vi "15-12-13 UHR-Fleezers Control (host) - 15.2.1UCB Darwin.vi"() -> ()   [LabVIEW 2014] (continued)
          tunnel: w1189 -> [_]
          tunnel: "Center Y Frequency (MHz)" -> [w1283]
          shift-right: [w1244] -> _
          shift-left: w1184 -> [w1251]
          shift-right: [w1242] -> _
          shift-left: w1184 -> [w1250]
          shift-right: [w1235] -> _
          shift-left: w1184 -> [w1248]
          shift-right: [w1233] -> _
          shift-left: w1184 -> [w1247]
          tunnel: "Move in a Circle" -> [_]
          tunnel: ["Back to start on finish?"] -> w1188
          tunnel: w1186 -> [_]
          tunnel: w1185 -> [w1265]
          tunnel: w1184 -> [w1246]
          shift-right: [w1217] -> _
          shift-left: 0.0 -> [w1215]
          i -> [w1224]
          stop <- w1288 stop-if-true
          w1232 = 0 ("index")
          w1253 = 1 ("dimension size")
          # "Keep phase within\n2pi so errors don't \nbuild"
          # "Accumulated\nphase"
          # "Current phase"
          # "Trap 2"
          # "Trap 1"
          # "ignore if N = 0"
          # "r"
          # "r"
          # "r"
          # "r"
          # "\"omega*t\""
          # "Trap 2"
          # "Trap separation (radians)"
          # "Trap 1"
          # "Offset (starts\n at bottom of\n the circle)"
          # "omega"
          n764 = node-c288() -> (w1301:i64)  [unwired: 1 in]
          n765 = Divide(x=w1301, y=1000) -> (x/y=w1220:dbl)
          n766 = Divide(x="2D Motion Trap Separation (MHz)", y="Radius (MHz)") -> (x/y=w1275:dbl)
          n767 = Negate(x=w1220) -> (-x=w1219:dbl)
          n768 = Divide(x="Trap 2 phase shift (deg)", y=360.0) -> (x/y=w1266:dbl)
          n769 = Inverse Sine(1:w1275) -> (0:w1211:dbl)
          n770 = Multiply(x=6.283185307179586, y=w1266) -> (x*y=w1212:dbl)
          n771 = Multiply(x=6.283185307179586, y="2D Motion Frequency (Hz)") -> (x*y=w1223:dbl)
          n772 = Select(t=w1220, s="Counterclockwise/Clockwise", f=w1219) -> (s? t:f=w1222:dbl)
          n773 = Multiply(x=w1223, y=w1222) -> (x*y=w1213:dbl)
          n774 = Select(t=w1211, s="Trap shift\nmethod", f=w1212) -> (s? t:f=w1210:dbl)
          n775 = Add(x=w1213, y=w1215) -> (x+y=w1216:dbl)
          n776 = Add(x=w1216, y=w1210) -> (x+y=w1272:dbl)
          n777 = Add(x=w1216, y=1.5707963267948966) -> (x+y=w1221:dbl)
          n778 = Add(x=w1272, y=1.5707963267948966) -> (x+y=w1285:dbl)
          n779 = Cosine(x=w1221) -> (cos(x)=w1299:dbl)
          n780 = Sine(x=w1221) -> (sin(x)=w1298:dbl)
          n781 = Multiply(x=w1299, y="Radius (MHz)") -> (x*y=w1292:dbl)
          n782 = Cosine(x=w1285) -> (cos(x)=w1297:dbl)
          n783 = Sine(x=w1285) -> (sin(x)=w1296:dbl)
          n784 = Multiply(x=w1298, y="Radius (MHz)") -> (x*y=w1291:dbl)
          n785 = Multiply(x=w1297, y="Radius (MHz)") -> (x*y=w1295:dbl)
          n786 = Multiply(x=w1296, y="Radius (MHz)") -> (x*y=w1293:dbl)
          n787 = Add(x=w1292, y=w1290) -> (x+y=w1241:dbl)
          n788 = Add(x=w1291, y=w1283) -> (x+y=w1239:dbl)
          n789 = Greater Or Equal?(x=w1224, y="N steps then stop") -> (x >= y?=w1282:bool)
          n790 = Add(x=w1295, y=w1294) -> (x+y=w1230:dbl)
          n791 = Add(x=w1293, y=w1283) -> (x+y=w1228:dbl)
          n792 = Not Equal To 0?(x="N steps then stop") -> (x != 0?=w1278:bool)
          n793 = And(x=w1282, y=w1278) -> (x .and. y?=w1279:bool)
          n794 = local read "Trap 1 sum mean"() -> (w1262:dbl)
          n795 = local read "Stop All"() -> (w1287:bool)
          n796 = local write "BD 1 Frequency 1 (MHz)"(w1241) -> ()
          n797 = local write "BD 2 Frequency 1 (MHz)"(w1239) -> ()
          n798 = local write "BD 1 Frequency 2 (MHz)"(w1230) -> ()
          n799 = local write "BD 2 Frequency 2 (MHz)"(w1228) -> ()
          n800 = Select(t=w1224, s="test", f=w1262) -> (s? t:f=→"Waveform Chart":dbl)
          n801 = Compound Arithmetic op=OR(w1287, "Stop Moving", w1279) -> (w1288:bool)
          n802 = local read "BD 1 Frequency 3 (MHz)"() -> (w1271:dbl)
          n803 = local read "BD 2 Frequency 3 (MHz)"() -> (w1270:dbl)
          n804 = Select(t=w1246, s="Reset graph", f=w1247) -> (s? t:f=w1227:dbl[])
          n805 = Select(t=w1246, s="Reset graph", f=w1248) -> (s? t:f=w1229:dbl[])
          n806 = Select(t=w1246, s="Reset graph", f=w1250) -> (s? t:f=w1238:dbl[])
          n807 = Select(t=w1246, s="Reset graph", f=w1251) -> (s? t:f=w1240:dbl[])
          n808 = Initialize Array(w1228, w1253) -> (w1254:dbl[])
          n809 = Initialize Array(w1239, w1253) -> (w1257:dbl[])
          n810 = Initialize Array(w1230, w1253) -> (w1255:dbl[])
          n811 = Initialize Array(w1241, w1253) -> (w1258:dbl[])
          n812 = local read "Y RF Frequency Limits (MHz)"() -> (w1268:T18)
          n813 = local read "X RF Frequency Limits (MHz)"() -> (w1269:T18)
          n814 = call "set RF board frequency - interlace.vi"("Board 2 Frequency Limits"=w1268, "Board 1 Frequency Limits"=w1269, "FPGA VI Reference In"=w1265, "Board 2 Frequency 3 (MHz)"=w1270, "Board 1 Frequency 3 (MHz)"=w1271, "Board 2 Frequency 2 (MHz)"=w1228, "Board 2 Frequency 1 (MHz)"=w1239, "Board 1 Frequency 2 (MHz)"=w1230, "Board 1 Frequency 1  (MHz)"=w1241) -> ()  [unwired: 1 in, 2 out]
          n815 = Bundle(w1255, w1254) -> (w1226:cluster{dbl[], dbl[]})  [unwired: 1 in]
          n816 = Bundle(w1258, w1257) -> (w1256:cluster{dbl[], dbl[]})  [unwired: 1 in]
          n817 = Build Array (concatenate)(w1241, w1240) -> (w1245:dbl[])
          n818 = Build Array (concatenate)(w1239, w1238) -> (w1243:dbl[])
          n819 = Build Array (concatenate)(w1230, w1229) -> (w1236:dbl[])
          n820 = Build Array (concatenate)(w1228, w1227) -> (w1234:dbl[])
          n821 = Bundle(w1245, w1243) -> (w1225:cluster{dbl[], dbl[]})  [unwired: 1 in]
          n822 = Bundle(w1236, w1234) -> (w1252:cluster{dbl[], dbl[]})  [unwired: 1 in]
          n823 = Build Array(w1256, w1226, w1225, w1252) -> (→"Trap trajectories":cluster{dbl[], dbl[]}[])
          n824 = case "To pause the process" shown="True" "Pause rotation" {
            frame False {
            }
            frame True {
              n825 = while {
                stop <- w1304 stop-if-true
                n826 = local read "Pause rotation"() -> (w1305:bool)
                n827 = Wait (ms)(milliseconds to wait=u32 10) -> ()  [unwired: 1 out]
                n828 = Not(x=w1305) -> (.not. x?=w1304:bool)
              }
            }
          }
          n829 = Decrement(x="N steps to plot") -> (x-1=w1231:i32)
          n830 = Array Subset(array=w1243, index=w1232, length=w1231) -> (w1242:dbl[])
          n831 = Array Subset(array=w1245, index=w1232, length=w1231) -> (w1244:dbl[])
          n832 = Array Subset(array=w1236, index=w1232, length=w1231) -> (w1235:dbl[])
          n833 = Array Subset(array=w1234, index=w1232, length=w1231) -> (w1233:dbl[])
          n834 = Quotient & Remainder(x=w1216, y=6.283185307179586) -> (x-y*floor(x/y)=w1217:dbl)  [unwired: 1 out]
          n835 = node-c288() -> ()  [unwired: 1 in, 1 out]
        }
        n836 = node-c288(w1197) -> ()  [unwired: 1 out]
        n837 = case shown="True" w1188 {
          tunnel: w1192 -> [_ w1203]
          tunnel: w1191 -> [_ w1202]
          tunnel: w1190 -> [_ w1201]
          tunnel: w1189 -> [_ w1200]
          frame False {
          }
          frame True {
            n838 = flat-sequence {
              tunnel: w1203 -> [w1207]
              tunnel: w1202 -> [w1206]
              tunnel: w1201 -> [w1205]
              tunnel: w1200 -> [w1204]
              frame #0 {
                n839 = local write "BD 1 Frequency 1 (MHz)"(w1207) -> ()
                n840 = local write "BD 2 Frequency 1 (MHz)"(w1206) -> ()
                n841 = local write "BD 1 Frequency 2 (MHz)"(w1205) -> ()
                n842 = local write "BD 2 Frequency 2 (MHz)"(w1204) -> ()
              }
              frame #1 {
                n843 = property on="Update all trap values" class="Bool (strict)"("Val(Sgnl)"=TRUE ("Value (Signaling)")) -> ()  [unwired: 2 in, 2 out]
              }
            }
          }
        }
      }
      event "Stop All": Value Change {
        # "Stopping blue laser before shutting off program"
        n844 = event-data() -> ()  [unwired: 1 in, 5 out]
        n845 = local read "Delay (ms)"() -> (w1315:i32)
        n846 = call "serial write macro.vi"("String"="l0", "Delay (ms)"=w1315, "VISA resource name"=w1318) -> ("read buffer"=w1313:string, "error out"=w1314:errorcluster, "VISA resource name out"=w1317:refnum<visa-resource-name>)
        n847 = local write "read blue buffer"(w1313) -> ()
        n848 = local write "Blue Error Out"(w1314) -> ()
        n849 = VISA Close(VISA resource name=w1317) -> ()  [unwired: 1 in, 1 out]
        n850 = local read "Stop All"() -> (w1319:bool)
      }
      event "Sensitivity", "Offset Current Sign", "Offset Current Value", "Offset Current", "Bias Voltage", "Bias Voltage (mV)", "Filter Type", "Lowpass 3dB Point", "Highpass 3dB Point", "Filter Reset", "Invert Signal", "Gain Mode", "Send Command": Value Change {
        w1326 = 250 ("Delay (ms)")
        n851 = event-data() -> ()  [unwired: 1 in, 5 out]
        n852 = event shown="[0] \"Sensitivity\": Value Change" {
          selector: _ -> [_ _ _ _ _ _ _ _ _ _ _ _ _]
          dyn-events: _ -> [_ _ _ _ _ _ _ _ _ _ _ _ _]
          timeout: _ -> [_ _ _ _ _ _ _ _ _ _ _ _ _]
          tunnel: [w1338 w1346 w1354 w1363 w1373 w1381 w1384 w1388 w1391 w1394 w1397 w1404 "Command"] -> w1325
          tunnel: [w1333 w1340 w1350 w1357 w1367 w1377 _ _ _ _ _ w1400 _] -> w1320
          event "Sensitivity": Value Change {
            n853 = event-data() -> ()  [unwired: 1 in, 5 out]
            n854 = property on="Sensitivity" class="CmbBox"() -> ("Value"=→"Gain":string)  [unwired: 2 in, 2 out]
            n855 = Concatenate Strings("SENS ", "Sensitivity") -> (w1338:string)
            n856 = local read "Gain"() -> (w1335:string)
            n857 = Concatenate Strings("gain set at ", w1335) -> (w1333:string)
          }
          event "Offset Current Sign": Value Change {
            n858 = event-data() -> ()  [unwired: 1 in, 4 out]
            n859 = Boolean To (0,1)(Boolean="Offset Current Sign") -> (0, 1=w1349:i16)
            n860 = Select(t="positive", s="Offset Current Sign", f="negative") -> (s? t:f=w1341:string)
            n861 = Number To Decimal String(number=w1349) -> (decimal integer string=w1348:string)  [unwired: 1 in]
            n862 = Concatenate Strings("IOSN " ("string"), w1348) -> (w1346:string)
            n863 = Concatenate Strings("offset current sign ", w1341) -> (w1340:string)
          }
          event "Offset Current Value": Value Change {
            n864 = event-data() -> ()  [unwired: 1 in, 5 out]
            n865 = property on="Offset Current Value" class="CmbBox"() -> ("Value"=→"Read offset current":string)  [unwired: 2 in, 2 out]
            n866 = local read "Read offset current"() -> (w1351:string)
            n867 = Concatenate Strings("IOLV ", "Offset Current Value") -> (w1354:string)
            n868 = Concatenate Strings("offset current value ", w1351) -> (w1350:string)
          }
          event "Offset Current": Value Change {
            n869 = event-data() -> ()  [unwired: 1 in, 5 out]
            n870 = Boolean To (0,1)(Boolean="Offset Current") -> (0, 1=w1366:i16)
            n871 = Select(t="on", s="Offset Current", f="off") -> (s? t:f=w1358:string)
            n872 = Number To Decimal String(number=w1366) -> (decimal integer string=w1365:string)  [unwired: 1 in]
            n873 = Concatenate Strings("IOON " ("string"), w1365) -> (w1363:string)
            n874 = Concatenate Strings("offset current ", w1358) -> (w1357:string)
          }
          event "Bias Voltage": Value Change {
            n875 = event-data() -> ()  [unwired: 1 in, 5 out]
            n876 = Boolean To (0,1)(Boolean="Bias Voltage") -> (0, 1=w1374:i16)
            n877 = Number To Decimal String(number=w1374) -> (decimal integer string=w1375:string)  [unwired: 1 in]
            n878 = Select(t="on", s="Bias Voltage", f="off") -> (s? t:f=w1368:string)
            n879 = Concatenate Strings("BSON " ("string"), w1375) -> (w1373:string)
            n880 = Concatenate Strings("bias voltage", w1368) -> (w1367:string)
          }
          event "Bias Voltage (mV)": Value Change {
            n881 = event-data() -> ()  [unwired: 1 in, 5 out]
            n882 = Number To Decimal String(number="Bias Voltage (mV)") -> (decimal integer string=w1383:string)  [unwired: 1 in]
            n883 = Number To Fractional String(number="Bias Voltage (mV)") -> (F-format string=w1378:string)  [unwired: 3 in]
            n884 = Concatenate Strings("BSLV " ("string"), w1383) -> (w1381:string)
            n885 = Concatenate Strings("bias voltage value ", w1378) -> (w1377:string)
          }
          event "Filter Type": Value Change {
            n886 = event-data() -> ()  [unwired: 1 in, 5 out]
            n887 = Concatenate Strings("FLTT " ("string"), "Filter Type") -> (w1384:string)
          }
          event "Lowpass 3dB Point": Value Change {
            n888 = event-data() -> ()  [unwired: 1 in, 5 out]
            n889 = Concatenate Strings("LFRQ " ("string"), "Lowpass 3dB Point") -> (w1388:string)
          }
          event "Highpass 3dB Point": Value Change {
            n890 = event-data() -> ()  [unwired: 1 in, 5 out]
            n891 = Concatenate Strings("HFRQ " ("string"), "Highpass 3dB Point") -> (w1391:string)
          }
          event "Filter Reset": Value Change {
            n892 = event-data() -> ()  [unwired: 1 in, 5 out]
            n893 = Select(t="ROLD", s="Filter Reset", f="") -> (s? t:f=w1394:string)
          }
          event "Gain Mode": Value Change {
            n894 = event-data() -> ()  [unwired: 1 in, 5 out]
            n895 = Concatenate Strings("GNMD " ("string"), "Gain Mode") -> (w1397:string)
          }
          event "Invert Signal": Value Change {
            n896 = event-data() -> ()  [unwired: 1 in, 5 out]
            n897 = Boolean To (0,1)(Boolean="Invert Signal") -> (0, 1=w1407:i16)
            n898 = Number To Decimal String(number=w1407) -> (decimal integer string=w1406:string)  [unwired: 1 in]
            n899 = Concatenate Strings("INVT " ("string"), w1406) -> (w1404:string)
            n900 = Select(t="signal inverted", s="Invert Signal", f="signal not inverted") -> (s? t:f=w1400:string)
          }
          event "Send Command": Value Change {
            n901 = event-data() -> ()  [unwired: 1 in, 5 out]
          }
        }
        "Command Sent" <- w1325
        n902 = local read "Save Event Log?"() -> (w1321:bool)
        n903 = local read "Saving..."() -> (w1322:bool)
        n904 = And(x=w1321, y=w1322) -> (x .and. y?=w1323:bool)
        n905 = case shown="True" w1323 {
          tunnel: w1320 -> [_ w1330]
          frame False {
          }
          frame True {
            n906 = local read "Time (s)"() -> (w1331:dbl)
            n907 = local read "log file ref"() -> (w1332:refnum<file>)
            n908 = call "write to event log.vi"("log file ref"=w1332, "time"=w1331, "input string"=w1330) -> ()  [unwired: 8 in]
          }
        }
        n909 = call "preamp serial write macro.vi"("String"=w1325, "Delay (ms)"=w1326, "VISA resource name"=w1329) -> ("read buffer"=→"Reply":string, "error out"=w1328:errorcluster)  [unwired: 1 out]
        n910 = call "preamp serial write macro.vi"("String"=w1325, "Delay (ms)"=w1326, "VISA resource name"=w1324) -> ()  [unwired: 3 out]
        n911 = local write "Preamp Error Out"(w1328) -> ()
      }
    }
    n912 = node-c288() -> ()  [unwired: 1 in, 1 out]
  }
  n913 = node-c288() -> (w27:T27)  [unwired: 4 out]
  n914 = node-c288(2 ("Processor")) -> (w59:T27)  [unwired: 3 out]
  n915 = disable-structure shown="Disabled" {
    frame Disabled {
      n916 = while "Duncan's play event loop" {
        stop <- w1411 stop-if-true
        n917 = Create User Event(user event datatype=TRUE ("Boolean")) -> (user event=w1412:refnum<user-event>)  [unwired: 1 in, 1 out]
        n918 = Create User Event(user event datatype=TRUE ("Boolean")) -> (user event=w1418:refnum<user-event>)  [unwired: 1 in, 1 out]
        n919 = global write "Global for fluorescence simulation mean (30 samples), (power series).vi" "Red Signal"(w1412) -> ()
        n920 = global write "Global for fluorescence simulation mean (30 samples), (power series).vi" "Green Signal"(w1418) -> ()
        n921 = register-events(w1418, w1412) -> (reference out=w1417:refnum<event-registration>)  [unwired: 2 in, 1 out]
        n922 = event shown="[1] \"Start assembly line\": Value Change" {
          selector: w1417 -> [_ _ _ _]
          dyn-events: _ -> [_ _ _ _]
          timeout: 100 -> [_ _ _ _]
          event Timeout {
            n923 = event-data() -> ()  [unwired: 1 in, 2 out]
          }
          event "Start assembly line": Value Change {
            n924 = event-data() -> ("OldVal"=w1420:bool)  [unwired: 1 in, 4 out]
            n925 = case shown="True" w1420 {
              selector: w1420 -> [_ w1421]
              frame False {
              }
              frame True {
                n926 = property on="Move to Position 3" class="Bool"("Val(Sgnl)"=w1421) -> ()  [unwired: 2 in, 2 out]
                n927 = case shown="1" "Numeric" {
                  frame 0, Default {
                  }
                  frame 1 {
                    n928 = property on="Green Laser ON" class="Bool (strict)"("Val(Sgnl)"=TRUE ("Value (Signaling)")) -> ()  [unwired: 2 in, 2 out]
                  }
                  frame 2 {
                    n929 = property on="Red Laser ON" class="Bool (strict)"("Val(Sgnl)"=TRUE) -> ()  [unwired: 2 in, 2 out]
                  }
                }
              }
            }
          }
          event User Event {
            n930 = event-data() -> ("Boolean"=w1425:bool)  [unwired: 1 in, 3 out]
            "Green Fluorophore" <- w1425
            n931 = property on="Start assembly line" class="Bool"("Val(Sgnl)"=w1425) -> ()  [unwired: 2 in, 2 out]
          }
          event User Event {
            n932 = event-data() -> ("Boolean"=w1426:bool)  [unwired: 1 in, 3 out]
            "Red Fluorophore" <- w1426
            n933 = property on="Start assembly line" class="Bool"("Val(Sgnl)"=w1426) -> ()  [unwired: 2 in, 2 out]
          }
        }
        n934 = property on="Get Fluorophore" class="Bool (strict)"("Val(Sgnl)"="Get Fluorophore") -> ()  [unwired: 2 in, 2 out]
        n935 = Wait (ms)(milliseconds to wait=u32 100) -> ()  [unwired: 1 out]
        n936 = local read "Stop All"() -> (w1410:bool)
        n937 = Or(x=w1410, y="stop") -> (x .or. y?=w1411:bool)
      }
    }
    frame Enabled {
    }
  }
  n938 = timed-loop "Rough control of MCL mirror stage (debugging)" {
    tunnel: [w1429] -> w68
    timing: w27 -> [_]
    timing-out: [_] -> w26
    tunnel: w15 -> [w1427]
    stop <- w1429 stop-if-true
    n939 = node-c288() -> ()  [unwired: 2 out]
    n940 = case shown="2" "MCL Mode" {
      tunnel: w1427 -> [_ w1432 w1479]
      frame 0, Default {
      }
      frame 1 {
        n941 = node-c288() -> (w1434:T27)  [unwired: 4 out]
        n942 = timed-loop "Oscillate MCL mirror" {
          timing: w1434 -> [_]
          timing-out: [_] -> w1433
          tunnel: w1432 -> [w1435]
          i -> [w1473]
          stop <- w1436 stop-if-true
          n943 = node-c288() -> (w1472:i64)  [unwired: 1 out]
          n944 = Multiply(x="AO1", y=32767.0) -> (x*y=w1468:dbl)
          n945 = Multiply(x="AO2", y=32767.0) -> (x*y=w1463:dbl)
          n946 = Divide(x=w1468, y=10.0) -> (x/y=w1469:dbl)
          n947 = Divide(x=w1463, y=10.0) -> (x/y=w1464:dbl)
          n948 = To Word Integer(number=w1469) -> (16bit integer=w1461:i16)
          n949 = To Word Integer(number=w1464) -> (16bit integer=w1460:i16)
          n950 = Divide(x=w1472, y=i64 1000) -> (x/y=w1443:dbl)
          n951 = Multiply(x=w1443, y=w1473) -> (x*y=w1454:dbl)
          n952 = Multiply(x="Osc. freq. (Hz) 2", y=6.283185307179586) -> (x*y=w1455:dbl)
          n953 = Multiply(x=w1455, y=w1454) -> (x*y=w1453:dbl)
          n954 = Sine(x=w1453) -> (sin(x)=w1452:dbl)
          n955 = Multiply(x=w1452, y="Osc. amp. (V)") -> (x*y=w1450:dbl)
          n956 = Add(x=w1450, y="Osc. center (V)") -> (x+y=w1448:dbl)
          n957 = Divide(x=w1448, y=10.0) -> (x/y=w1446:dbl)
          n958 = Multiply(x=w1446, y=32767.0) -> (x*y=w1441:dbl)
          n959 = Select(t=w1441, s="Scan axis", f=w1461) -> (s? t:f=w1459:dbl)
          n960 = Select(t=w1460, s="Scan axis", f=w1441) -> (s? t:f=w1458:dbl)
          n961 = local read "MCL Mode"() -> (w1440:u16)
          n962 = Not Equal?(x=w1440, y=u16 1) -> (x != y?=w1437:bool)
          n963 = local read "Stop All"() -> (w1438:bool)
          n964 = xnode "Read/Write Control"("FPGA VI Reference In"=w1435, "AO1"=w1459, "AO2"=w1458) -> ()  [unwired: 1 in, 2 out]
          n965 = Compound Arithmetic op=OR(w1438, w1437) -> (w1436:bool)
          n966 = node-c288() -> ()  [unwired: 2 out]
        }
        n967 = node-c288(w1433) -> ()  [unwired: 1 out]
      }
      frame 2 {
        n968 = case shown="True" "Start Scan" {
          tunnel: w1479 -> [_ w1481]
          frame False {
          }
          frame True {
            n969 = Subtract(x="End (V)", y="Begin (V)") -> (x-y=w1488:dbl)
            n970 = Decrement(x="N Points") -> (x-1=w1487:dbl)
            n971 = Divide(x=w1488, y=w1487) -> (x/y=w1485:dbl)
            n972 = for {
              N: "N Points" -> [_]
              tunnel: "Begin (V)" -> [w1504]
              tunnel: [w1496] -> w1491 mode=indexing
              tunnel: w1485 -> [w1495]
              tunnel: [w1493] -> w1484 mode=indexing
              tunnel: w1481 -> [w1492]
              i -> [w1503]
              n973 = Multiply(x=w1495, y=w1503) -> (x*y=w1502:dbl)
              n974 = Add(x=w1504, y=w1502) -> (x+y=w1499:dbl)
              n975 = local read "Scan axis"() -> (w1494:bool)
              n976 = local read "AO1"() -> (w1501:dbl)
              n977 = local read "AO2"() -> (w1500:dbl)
              n978 = Select(t=w1499, s=w1494, f=w1501) -> (s? t:f=w1498:dbl)
              n979 = Select(t=w1500, s=w1494, f=w1499) -> (s? t:f=w1497:dbl)
              n980 = flat-sequence {
                tunnel: w1498 -> [w1508]
                tunnel: w1497 -> [w1507]
                tunnel: w1492 -> [w1505]
                tunnel: [w1518] -> w1496
                tunnel: [w1517] -> w1493
                frame #0 {
                  w1511 = 10.0 ("y")
                  w1506 = 32767.0 ("y")
                  n981 = Multiply(x=w1508, y=w1506) -> (x*y=w1514:dbl)
                  n982 = Multiply(x=w1507, y=w1506) -> (x*y=w1512:dbl)
                  n983 = Divide(x=w1514, y=w1511) -> (x/y=w1515:dbl)
                  n984 = Divide(x=w1512, y=w1511) -> (x/y=w1513:dbl)
                  n985 = To Word Integer(number=w1515) -> (16bit integer=w1509:i16)
                  n986 = To Word Integer(number=w1513) -> (16bit integer=w1510:i16)
                  n987 = xnode "Read/Write Control"("FPGA VI Reference In"=w1505, "AO1"=w1509, "AO2"=w1510) -> ()  [unwired: 1 in, 2 out]
                }
                frame #1 {
                  n988 = Wait (ms)(milliseconds to wait="DAQ Delay (ms)") -> ()  [unwired: 1 out]
                }
                frame #2 {
                  n989 = local read "Slow mean"() -> (w1518:dbl)
                  n990 = local read "Sigma"() -> (w1517:dbl)
                }
              }
            }
            n991 = Bundle("Begin (V)"="Begin (V)", w1485, w1491) -> (→"MCL Scan":cluster{"Begin (V)":dbl, dbl, dbl[]})  [unwired: 1 out]
            n992 = Bundle("Begin (V)"="Begin (V)", w1485, w1484) -> (→"MCL Scan 2":cluster{"Begin (V)":dbl, dbl, dbl[]})  [unwired: 1 out]
          }
        }
      }
    }
    n993 = local read "Stop All"() -> (w1429:bool)
    n994 = node-c288() -> ()  [unwired: 2 out]
  }
  n995 = timed-loop "Basic control parameters (all FPGA settings, other basic controls)" {
    shift-right: [w1526] -> _
    shift-left: errorcluster {"status"=FALSE, "code"=0, "source"=""} ("error out") -> [_]
    tunnel: [w1525] -> _
    timing: w59 -> [_]
    timing-out: [_] -> w58
    tunnel: w40 -> [w1524]
    tunnel: w36 -> [w1523]
    tunnel: w35 -> [w1522]
    tunnel: w34 -> [w1521]
    tunnel: w33 -> [w1520]
    tunnel: w15 -> [w1519]
    stop <- w1525 stop-if-true
    n996 = node-c288() -> ()  [unwired: 2 out]
    n997 = event shown="[25] \"+ phase (APD 1 Gate)\", \"- phase (APD 1 Gate)\", \"+ phase (APD 2 Gate)\", \"- phase (APD 2 Gate)\", \"+ phase (APD 3 Gate)\", \"- phase (APD 3 Gate)\", \"+ phase (APD Acq)\", \"- phase (APD Acq)\": Value Change" {
      selector: _ -> [_ _ _ _ _ _ _ _ _ _ _ _ _ _ _ _ _ _ _ _ _ _ _ _ _ _ _ _ _ _ _ _ _ _ _ _ _ _ _ _ _ _ _ _ _ _ _ _ _ _ _ _ _ _ _ _ _ _ _ _ _ _ _ _ _ _ _ _ _ _ _ _ _ _ _ _ _ _]
      dyn-events: _ -> [_ _ _ _ _ _ _ _ _ _ _ _ _ _ _ _ _ _ _ _ _ _ _ _ _ _ _ _ _ _ _ _ _ _ _ _ _ _ _ _ _ _ _ _ _ _ _ _ _ _ _ _ _ _ _ _ _ _ _ _ _ _ _ _ _ _ _ _ _ _ _ _ _ _ _ _ _ _]
      timeout: _ -> [_ _ _ _ _ _ _ _ _ _ _ _ _ _ _ _ _ _ _ _ _ _ _ _ _ _ _ _ _ _ _ _ _ _ _ _ _ _ _ _ _ _ _ _ _ _ _ _ _ _ _ _ _ _ _ _ _ _ _ _ _ _ _ _ _ _ _ _ _ _ _ _ _ _ _ _ _ _]
      tunnel: [w1566 _ _ _ w1596 _ _ _ _ _ _ w1667 _ _ w1755 w1757 w1766 w1768 w1838 _ w1880 w1906 w1934 w1959 w1986 w2012 w2041 _ w2046 w2140 w2144 w2181 _ w2219 w2222 w2225 w2235 w2238 _ w2245 _ _ _ _ _ _ _ _ _ _ _ _ _ _ _ _ _ w2709 _ _ _ _ w2745 _ _ _ _ _ _ _ _ _ _ _ _ _ _ _] -> w1526
      tunnel: [_ _ _ _ _ _ _ _ _ w1652 _ _ _ _ _ _ _ _ _ _ _ _ _ _ _ _ _ _ _ _ _ _ _ _ _ _ _ _ _ _ _ _ _ _ _ _ _ _ _ _ _ _ _ _ _ _ _ _ _ _ _ _ _ _ _ _ _ _ _ _ _ _ _ _ _ _ _ _] -> w1525
      tunnel: [_ _ _ _ _ _ _ "Round T1 X" _ _ _ _ _ _ _ _ _ _ _ _ _ _ _ _ _ _ _ _ _ _ _ _ _ _ _ _ _ _ _ _ _ _ _ _ _ _ _ _ _ _ _ _ _ _ _ _ _ _ _ _ _ _ _ _ _ _ _ _ _ _ _ _ _ _ _ _ _ _] -> _
      tunnel: [_ _ _ "Adjust Scale\nto Mean" _ _ _ _ _ _ _ _ _ _ _ _ _ _ _ _ _ _ _ _ _ _ _ _ "Test ttrig" _ _ _ _ _ _ _ _ _ _ _ _ _ _ _ _ _ _ "Flush Sample" "Flush Pump 3" "Flush Pump 1" "Clear Volume" _ _ _ _ _ _ _ _ _ _ _ _ _ _ _ _ _ _ _ _ _ _ _ _ _ _ _] -> _
      tunnel: [_ _ _ _ _ _ _ _ "Round T2 X" _ "Delayed Interlace Start" _ _ _ _ _ _ _ _ _ _ _ _ _ _ _ _ _ _ _ _ _ _ _ _ _ _ _ _ _ _ _ _ _ _ _ _ _ _ _ _ _ _ _ _ _ _ _ _ _ _ _ _ _ _ _ _ _ _ _ _ _ _ _ _ _ _ _] -> _
      tunnel: w1524 -> [_ _ _ _ _ _ _ _ _ _ _ _ _ _ _ _ _ _ _ _ _ _ _ _ _ _ _ _ _ _ _ _ _ _ _ _ _ _ _ _ _ _ _ w2444 w2451 w2458 w2463 w2477 _ _ w2623 _ _ _ _ _ _ _ _ _ _ _ _ _ _ _ _ _ _ _ _ _ _ _ _ _ _ _]
      tunnel: w1523 -> [_ _ _ _ _ _ _ _ _ _ _ _ _ _ _ _ _ _ _ _ _ _ _ _ _ _ _ _ _ _ _ _ _ _ _ _ _ _ _ _ _ w2333 _ _ _ _ _ _ w2536 _ _ w2629 _ w2638 _ w2652 _ _ _ _ _ _ _ _ _ _ _ _ _ _ _ _ _ _ _ _ _ _]
      tunnel: w1522 -> [_ _ _ _ _ _ _ _ _ _ _ _ _ _ _ _ _ _ _ _ _ _ _ _ _ _ _ _ _ _ _ _ _ _ _ _ _ _ _ _ _ _ _ _ _ _ _ _ _ _ _ _ _ _ _ _ _ _ _ _ _ _ _ _ _ _ _ _ _ _ _ _ _ _ _ _ _ _]
      tunnel: w1521 -> [_ _ _ _ _ _ _ _ _ _ _ _ _ _ _ _ _ _ _ _ _ _ _ _ _ _ _ _ _ _ _ _ _ _ _ _ _ _ _ _ w2256 _ _ _ _ _ _ _ _ w2581 _ _ w2634 _ w2645 _ w2677 _ _ _ _ _ _ _ _ _ _ _ _ _ _ _ _ _ _ _ _ _]
      tunnel: w1520 -> [_ _ _ _ _ _ _ _ _ _ _ _ _ _ _ _ _ _ _ _ _ _ _ _ _ _ _ _ _ _ _ _ _ _ _ _ _ _ _ _ _ _ _ _ _ _ _ _ _ _ _ _ _ _ _ _ _ _ _ _ _ _ _ _ _ _ _ _ _ _ _ _ _ _ _ _ _ _]
      tunnel: w1519 -> [w1529 _ _ _ w1595 _ w1621 _ _ _ _ w1658 _ _ w1736 w1756 w1761 w1767 w1803 _ w1869 w1904 w1916 w1941 w1969 w1989 w2017 w2042 w2044 w2048 w2141 w2145 _ w2216 w2220 w2223 w2233 w2236 _ w2244 _ _ _ _ _ _ _ _ _ _ _ _ _ _ _ _ _ w2702 _ w2723 _ w2729 w2744 _ w2751 w2753 w2760 w2774 w2789 _ w2798 _ w2818 _ _ w2872 w2905 w2906]
      event "AI Count (ticks)", "Sets to FIFO (Traps)", "Save ave N", "FPGA Ave.", "# Samples/channel", "N sets to save": Value Change {
        # "So that if 'Save ave N' is updated, the AOD scanning code updates too."
        n998 = event-data() -> ()  [unwired: 6 out]
        n999 = local read "AI Count (ticks)"() -> (w1550:u16)
        n1000 = Unbundle By Name("Sets to FIFO (Traps)") -> ("Set 1"=w1533:bool, "Set 2"=w1532:bool, "Set 3"=w1531:bool)
        n1001 = Boolean To (0,1)(Boolean="Sets to FIFO (Traps)") -> (0, 1=w1558:cluster{"Set 1":i16, "Set 2":i16, "Set 3":i16})
        n1002 = xnode "Read/Write Control"("FPGA VI Reference In"=w1529, "ai count"=w1550, "Set 1"=w1533, "Set 2"=w1532, "Set 3"=w1531, "N of AI1 Int Acq Sets"="N Acq Sets (Traps + Fl.)") -> ("error out"=w1566:errorcluster)  [unwired: 1 in, 1 out]
        n1003 = Cluster To Array(cluster=w1558) -> (array=w1557:i16[])
        n1004 = To Unsigned Long Integer(number=w1557) -> (unsigned 32bit integer=w1539:u32[])
        n1005 = local read "Scan steps (AOD)"() -> (w1559:u64)
        n1006 = Multiply(x=w1550, y="N Acq Sets (Traps + Fl.)") -> (x*y=w1548:u16)
        n1007 = Divide(x=40000000.0, y=w1550) -> (x/y=w1542:dbl)
        "AI rate (Hz)" <- w1542
        "Ave. Rate (Hz)" <- w1542
        n1008 = Add Array Elements(numeric array=w1539) -> (sum=w1551:u32)
        "Trap Sets" <- w1551
        n1009 = Reciprocal(x=w1542) -> (1/x=→"Ave. Period (s)":dbl)
        n1010 = property on="Scan steps (AOD)" class="DigNum (strict)"("Val(Sgnl)"=w1559) -> ()  [unwired: 2 in, 2 out]
        n1011 = Divide(x=w1542, y="N Acq Sets (Traps + Fl.)") -> (x/y=w1563:dbl)
        "Data Rate (Hz)" <- w1563
        n1012 = Reciprocal(x=w1563) -> (1/x=→"Data Period (s)":dbl)
        n1013 = local read "Save ave N"() -> (w1562:dbl)
        n1014 = Divide(x=w1563, y=w1562) -> (x/y=w1561:dbl)
        "Save Data Rate (Hz)" <- w1561
        n1015 = Reciprocal(x=w1561) -> (1/x=→"Save Data Period (s)":dbl)
        n1016 = Multiply(x=w1548, y="# Samples/trap") -> (x*y=w1546:u32)
        "Counts/DMA" <- w1546
        n1017 = property on="Trap Disp. Downsample" class="DigNum (strict)"("Maximum"="# Samples/trap") -> ()  [unwired: 2 in, 2 out]
        n1018 = Multiply(x=w1551, y="# Samples/trap") -> (x*y=w1540:u32)
        "# Samples/channel" <- w1540
        n1019 = Multiply(x=w1540, y=u32 8) -> (x*y=→"Trap AI Elements/DMA read":u32)
        n1020 = local read "APD Int. Count"() -> (w1547:u32)
        n1021 = Multiply(x=w1540, y=u32 3) -> (x*y=→"Trap Pos Elements/DMA read":u32)
        n1022 = Divide(x=w1546, y=w1547) -> (x/y=w1537:dbl)
        "APD Samples/FIFO Acq." <- w1537
        n1023 = Divide(x=w1546, y=40000000.0) -> (x/y=w1544:dbl)
        "DMA Update Period (s)" <- w1544
        n1024 = local read "Number of APDs"() -> (w1530:u8)
        n1025 = Multiply(x=w1530, y=w1537) -> (x*y=→"APD Elements/DMA read":dbl)
        n1026 = property on="APD Disp. Downsample" class="DigNum (strict)"("Maximum"=w1537) -> ()  [unwired: 2 in, 2 out]
        n1027 = local read "N sets to save"() -> (w1556:u32)
        n1028 = Multiply(x=w1544, y=w1556) -> (x*y=→"Total Time (s) 2":dbl)
        "FPGA Averaging" <- FALSE ("FPGA Averaging")
      }
      event "Remove Offset": Value Change {
        n1029 = event-data() -> ()  [unwired: 7 out]
        n1030 = local write "Remove Offset"(FALSE ("Remove Offset")) -> ()
        n1031 = local read "Bead Mean (nm)"() -> (w1568:dbl)
        n1032 = local read "Offset (nm)"() -> (w1569:dbl)
        n1033 = Add(x=w1568, y=w1569) -> (x+y=w1567:dbl)
        n1034 = local write "Offset (nm)"(w1567) -> ()
        n1035 = disable-structure shown="Disabled" {
          frame Disabled {
            n1036 = local read "Bead Mean (nm)"() -> (w1574:dbl)
            n1037 = Add(y=w1574) -> (x=w1573:dbl, x+y=w1572:dbl)
            n1038 = Subtract(x=w1574, y=w1573) -> (x-y=w1571:dbl)
            n1039 = property on="Bead Separation" class="WFChart (strict)"("YScale.Minimum"=w1571) -> ()  [unwired: 2 in, 2 out]
            n1040 = property on="Bead Separation" class="WFChart (strict)"("YScale.Maximum"=w1572) -> ()  [unwired: 2 in, 2 out]
          }
          frame Enabled {
          }
        }
      }
      event "Detector Type": Value Change {
        n1041 = event-data() -> ()  [unwired: 7 out]
        n1042 = local read "AI labels"() -> (w1576:string[])
        n1043 = property on="High Res. Display" class="Ring (strict)"("Strings []"=w1576) -> ()  [unwired: 2 in, 2 out]
        n1044 = Build Array (concatenate)(w1576, "none") -> (w1577:string[])
        n1045 = property on="FFT 1 Choice 1" class="Ring (strict)"("Strings []"=w1577) -> ()  [unwired: 2 in, 2 out]
        n1046 = property on="FFT 1 Choice 2" class="Ring (strict)"("Strings []"=w1577) -> ()  [unwired: 2 in, 2 out]
        n1047 = property on="FFT 2 Choice 1" class="Ring (strict)"("Strings []"=w1577) -> ()  [unwired: 2 in, 2 out]
        n1048 = property on="FFT 2 Choice 2" class="Ring (strict)"("Strings []"=w1577) -> ()  [unwired: 2 in, 2 out]
        n1049 = Bundle("APD 1", "APD 2", "APD 3") -> (w1580:cluster{string, string, string})  [unwired: 1 out]
        n1050 = Cluster To Array(cluster=w1580) -> (array=w1578:string[])
        n1051 = Build Array (concatenate)(w1578, w1577) -> (w1582:string[])
        n1052 = Array Size(array=w1582) -> (size(s)=w1583:i32)
        n1053 = property on="Signals to Plot" class="LstBox (strict)"("Item Names"=w1582) -> ()  [unwired: 2 in, 2 out]
        n1054 = property on="Signals to Plot" class="LstBox (strict)"("Number of Rows"=w1583) -> ()  [unwired: 2 in, 2 out]
        n1055 = property on="All Signals" class="WFChart (strict)"("LegNumRows"=w1583) -> ()  [unwired: 2 in, 2 out]
      }
      event "Adjust Scale\nto Mean": Value Change {
        n1056 = event-data() -> ()  [unwired: 7 out]
        n1057 = local read "APD 1 Rate (Hz)"() -> (w1592:dbl)
        n1058 = Multiply(x=1000.0, y="Above (kHz)") -> (x*y=w1590:dbl)
        n1059 = Multiply(x=1000.0, y="Below (kHz)") -> (x*y=w1588:dbl)
        n1060 = Add(x=w1590, y=w1592) -> (x+y=w1585:dbl)
        n1061 = Subtract(x=w1592, y=w1588) -> (x-y=w1586:dbl)
        n1062 = property on="APD Chart" class="WFChart (strict)"("YScale.Minimum"=w1586) -> ()  [unwired: 2 in, 2 out]
        n1063 = property on="APD Chart" class="WFChart (strict)"("YScale.Maximum"=w1585) -> ()  [unwired: 2 in, 2 out]
      }
      event "Phase adj. (AI1)", "+ phase (AI1)", "- phase (AI1)": Value Change {
        n1064 = event-data() -> ()  [unwired: 7 out]
        n1065 = Negate(x="Phase adj. (AI1)") -> (-x=w1603:i16)
        n1066 = Select(t=w1603, s="- phase (AI1)", f="Phase adj. (AI1)") -> (s? t:f=w1602:i16)
        n1067 = xnode "Read/Write Control"("FPGA VI Reference In"=w1595, "Phase count adjustment"=w1602) -> ("FPGA VI Reference Out"=w1601:T24, "error out"=w1600:errorcluster)  [unwired: 2 in]
        n1068 = Or(x="- phase (AI1)", y="+ phase (AI1)") -> (x .or. y?=w1597:bool)
        n1069 = xnode "Read/Write Control"("FPGA VI Reference In"=w1601, "error in"=w1600, "+ phase"=w1597) -> ("error out"=w1596:errorcluster)  [unwired: 1 in, 1 out]
      }
      event "Signals to Plot": Double Click {
        w1607 = u32 9868950 ("Color Box")
        n1070 = event-data() -> ("Row"=w1609:i32)  [unwired: 9 out]
        n1071 = property on="All Signals" class="WFChart (strict)"("Active Plot"=w1609) -> (error out=w1620:errorcluster)  [unwired: 2 in, 1 out]
        n1072 = property on="All Signals" class="WFChart (strict)" props=["Plot", "Visible?", "Plot", "Plot Color"](error in=w1620) -> (error out=w1619:errorcluster, "Plot.Visible?"=w1618:bool)  [unwired: 1 in, 2 out]
        n1073 = Select(t=FALSE ("Plot.Visible"), s=w1618, f=TRUE ("Plot.Visible")) -> (s? t:f=w1613:bool)
        n1074 = property on="All Signals" class="WFChart (strict)"(error in=w1619, "Plot.Visible?"=w1613) -> (error out=w1615:errorcluster)  [unwired: 1 in, 1 out]
        n1075 = property on="All Signals" class="WFChart (strict)"(error in=w1615) -> (error out=w1610:errorcluster, "Plot.Plot Color"=w1614:u32)  [unwired: 1 in, 1 out]
        n1076 = property on="Signals to Plot" class="LstBox (strict)"(error in=w1610, "Active Row"=w1609) -> (error out=w1608:errorcluster)  [unwired: 1 in, 1 out]
        n1077 = Select(t=w1614, s=w1613, f=u32 0) -> (s? t:f=w1611:u32)
        n1078 = property on="Signals to Plot" class="LstBox (strict)"(error in=w1608, "CellFontColor"=w1611, "SelColor"=w1607, "CellBG"=w1607, "CellFontSize"=u32 20 ("Active Row:Cell Font:Size"), "CellFontBold"=TRUE ("Active Row:Cell Font:Bold")) -> ()  [unwired: 1 in, 2 out]
      }
      event "BD 1 Frequency 1 (MHz)", "BD 1 Frequency 2 (MHz)", "BD 1 Frequency 3 (MHz)", "BD 2 Frequency 1 (MHz)", "BD 2 Frequency 2 (MHz)", "BD 2 Frequency 3 (MHz)", "Trap Delta (MHz)", "Update all trap values": Value Change {
        # "This is so you can set trap frequencies\nvia local variables and then update\nall at once"
        n1079 = event-data() -> ("CtlRef"=w1625:refnum<vi>)  [unwired: 6 out]
        n1080 = control-ref of="Trap Delta (MHz)"() -> (w1624:refnum<vi>)
        n1081 = Equal?(x=w1624, y=w1625) -> (x = y?=w1623:bool)
        n1082 = local write "Update all trap values"(FALSE ("Update all trap values")) -> ()
        n1083 = case shown="False" "Oscillate Set 1" {
          tunnel: w1623 -> [w1629 _]
          tunnel: w1621 -> [w1627 _]
          frame False {
            n1084 = local read "BD 1 Frequency 2 (MHz)"() -> (w1633:dbl)
            n1085 = local read "BD 1 Frequency 1 (MHz)"() -> (w1631:dbl)
            n1086 = Subtract(x=w1633, y="Trap Delta (MHz)") -> (x-y=w1630:dbl)
            n1087 = Select(t=w1630, s=w1629, f=w1631) -> (s? t:f=w1628:dbl)
            n1088 = local read "Y RF Frequency Limits (MHz)"() -> (w1634:T18)
            n1089 = local read "X RF Frequency Limits (MHz)"() -> (w1635:T18)
            n1090 = local write "BD 1 Frequency 1 (MHz)"(w1628) -> ()
            n1091 = local read "BD 1 Frequency 3 (MHz)"() -> (w1644:dbl)
            n1092 = local read "BD 2 Frequency 1 (MHz)"() -> (w1638:dbl)
            n1093 = local read "BD 2 Frequency 2 (MHz)"() -> (w1637:dbl)
            n1094 = local read "BD 2 Frequency 3 (MHz)"() -> (w1645:dbl)
            n1095 = call "set RF board frequency - interlace.vi"("Board 2 Frequency Limits"=w1634, "Board 1 Frequency Limits"=w1635, "FPGA VI Reference In"=w1627, "Board 2 Frequency 3 (MHz)"=w1645, "Board 1 Frequency 3 (MHz)"=w1644, "Board 2 Frequency 2 (MHz)"=w1637, "Board 2 Frequency 1 (MHz)"=w1638, "Board 1 Frequency 2 (MHz)"=w1633, "Board 1 Frequency 1  (MHz)"=w1628) -> ()  [unwired: 1 in, 2 out]
            n1096 = Subtract(x=w1638, y=w1637) -> (x-y=w1642:dbl)
            n1097 = Subtract(x=w1628, y=w1633) -> (x-y=w1643:dbl)
            n1098 = Square(x=w1642) -> (x^2=w1640:dbl)
            n1099 = Square(x=w1643) -> (x^2=w1641:dbl)
            n1100 = Add(x=w1641, y=w1640) -> (x+y=w1639:dbl)
            n1101 = Square Root(x=w1639) -> (sqrt(x)=w1636:dbl)
            n1102 = property on="Initial delta (MHz)" class="DigNum (strict)"("Val(Sgnl)"=w1636) -> ()  [unwired: 2 in, 2 out]
            n1103 = local write "Trap Delta (MHz)"(w1636) -> ()
          }
          frame True {
          }
        }
      }
      event "Round T1 X": Value Change {
        n1104 = event-data() -> ()  [unwired: 7 out]
        n1105 = local read "BD 1 Frequency 1 (MHz)"() -> (w1648:dbl)
        n1106 = Round To Nearest(number=w1648) -> (nearest integer value=w1647:dbl)
        n1107 = property on="BD 1 Frequency 1 (MHz)" class="DigNum (strict)"("Val(Sgnl)"=w1647) -> ()  [unwired: 2 in, 2 out]
      }
      event "Round T2 X": Value Change {
        n1108 = event-data() -> ()  [unwired: 7 out]
        n1109 = local read "BD 1 Frequency 2 (MHz)"() -> (w1650:dbl)
        n1110 = Round To Nearest(number=w1650) -> (nearest integer value=w1649:dbl)
        n1111 = property on="BD 1 Frequency 2 (MHz)" class="DigNum (strict)"("Val(Sgnl)"=w1649) -> ()  [unwired: 2 in, 2 out]
      }
      event "Stop All": Value Change {
        n1112 = event-data() -> ()  [unwired: 7 out]
        n1113 = local read "Stop All"() -> (w1652:bool)
      }
      event "Delayed Interlace Start": Value Change {
        n1114 = event-data() -> ()  [unwired: 7 out]
        n1115 = flat-sequence {
          frame #0 {
            n1116 = Multiply(x="Delay to Interlace (s)", y=1000.0) -> (x*y=w1654:dbl)
            n1117 = Wait (ms)(milliseconds to wait=w1654) -> ()  [unwired: 1 out]
          }
          frame #1 {
            n1118 = property on="Laser interlacing mode" class="RadioBtnsControl (strict)"("Val(Sgnl)"=enum32{"Laser ON", "Laser OFF", "Interlace"}."Interlace" ("Value (Signaling)")) -> ()  [unwired: 2 in, 2 out]
          }
        }
      }
      event "BD 1 Amplitude 1 (%)", "BD 1 Amplitude 2 (%)", "BD 1 Amplitude 3 (%)", "BD 2 Amplitude 1 (%)", "BD 2 Amplitude 2 (%)", "BD 2 Amplitude 3 (%)", "Trap 1 ON", "Trap 2 ON", "Trap 3 ON", "Feedback On/Off", "All FB On/Off": Value Change {
        w1679 = i16 1 ("f")
        n1119 = event-data() -> ()  [unwired: 7 out]
        n1120 = local write "Trap 1 (ON/OFF)"("Trap 1 ON") -> ()
        n1121 = local write "Trap 2 (ON/OFF)"("Trap 2 ON") -> ()
        n1122 = Boolean To (0,1)(Boolean="Trap 3 ON") -> (0, 1=w1680:i16)
        n1123 = Boolean To (0,1)(Boolean="Trap 1 ON") -> (0, 1=w1681:i16)
        n1124 = Boolean To (0,1)(Boolean="Trap 2 ON") -> (0, 1=w1682:i16)
        n1125 = Select(t=w1682, s="Trap ON/OFF X or Y Amp?", f=w1679) -> (s? t:f=w1677:i16)
        n1126 = Select(t=w1681, s="Trap ON/OFF X or Y Amp?", f=w1679) -> (s? t:f=w1678:i16)
        n1127 = Select(t=w1680, s="Trap ON/OFF X or Y Amp?", f=w1679) -> (s? t:f=w1676:i16)
        n1128 = Select(t=w1679, s="Trap ON/OFF X or Y Amp?", f=w1682) -> (s? t:f=w1674:i16)
        n1129 = Select(t=w1679, s="Trap ON/OFF X or Y Amp?", f=w1681) -> (s? t:f=w1675:i16)
        n1130 = Select(t=w1679, s="Trap ON/OFF X or Y Amp?", f=w1680) -> (s? t:f=w1673:i16)
        n1131 = And(x="All FB On/Off", y="Feedback On/Off") -> (x .and. y?=w1671:cluster{"Set 1":bool, "Set 2":bool})
        n1132 = local read "BD 1 Amplitude 1 (%)"() -> (w1689:dbl)
        n1133 = local read "BD 1 Amplitude 2 (%)"() -> (w1688:dbl)
        n1134 = local read "BD 1 Amplitude 3 (%)"() -> (w1687:dbl)
        n1135 = Unbundle By Name(w1671) -> ("Set 1"=w1666:bool, "Set 2"=w1663:bool)
        n1136 = local read "Y RF Amplitude Limits (%)"() -> (w1659:T18)
        n1137 = local read "X RF Amplitude Limits (%)"() -> (w1660:T18)
        n1138 = local read "BD 2 Amplitude 1 (%)"() -> (w1690:dbl)
        n1139 = local read "BD 2 Amplitude 2 (%)"() -> (w1691:dbl)
        n1140 = local read "BD 2 Amplitude 3 (%)"() -> (w1692:dbl)
        n1141 = And(x="Trap 2 ON", y=w1663) -> (x .and. y?=w1661:bool)
        n1142 = And(x="Trap 1 ON", y=w1666) -> (x .and. y?=w1664:bool)
        n1143 = Multiply(x=w1678, y=w1689) -> (x*y=w1686:dbl)
        n1144 = Multiply(x=w1688, y=w1677) -> (x*y=w1684:dbl)
        n1145 = Multiply(x=w1687, y=w1676) -> (x*y=w1685:dbl)
        n1146 = Multiply(x=w1690, y=w1675) -> (x*y=w1693:dbl)
        n1147 = Multiply(x=w1691, y=w1674) -> (x*y=w1694:dbl)
        n1148 = Multiply(x=w1692, y=w1673) -> (x*y=w1695:dbl)
        n1149 = call "set RF board amplitude - interlace.vi"("Board 2 Amplitude Limits"=w1659, "Board 1 Amplitude Limits"=w1660, "FPGA VI Reference In"=w1658, "Board 2 Amplitude 3 (%)"=w1695, "Board 1 Amplitude 3 (%)"=w1685, "Board 2 Amplitude 2 (%)"=w1694, "Board 2 Amplitude 1 (%)"=w1693, "Board 1 Amplitude 2 (%)"=w1684, "Board 1 Amplitude 1 (%)"=w1686) -> ("error out"=w1668:errorcluster, "FPGA VI Reference Out"=w1669:T24)  [unwired: 1 in]
        n1150 = xnode "Read/Write Control"("FPGA VI Reference In"=w1669, "error in"=w1668, "FB On/Off Set 1"=w1664, "FB On/Off Set 2"=w1661) -> ("error out"=w1667:errorcluster)  [unwired: 1 out]
      }
      event "Load parameters": Value Change {
        n1151 = event-data() -> ()  [unwired: 7 out]
        n1152 = property on="Saved AOD Raster Scan Parameter Sets" class="Arr (strict)"() -> ("Index Values"=w1706:u32[])  [unwired: 2 in, 2 out]
        n1153 = Index Array(array=w1706, index=0) -> (element=w1703:u32)
        n1154 = local write "Load parameters"(FALSE ("Load parameters")) -> ()
        n1155 = Index Array(array="Saved AOD Raster Scan Parameter Sets", index=w1703) -> (element=w1702:T34)
        n1156 = Unbundle By Name(w1702) -> ("Scan Range AOD (nm) 2"=w1701:dbl, "Step Size AOD (nm) 2"=w1700:dbl, "Scan Speed AOD (nm/s) 2"=w1699:dbl, "Number of scans (AOD) 2"=w1698:u16)
        n1157 = flat-sequence {
          tunnel: w1701 -> [w1709]
          tunnel: w1700 -> [w1708]
          tunnel: w1699 -> [w1707]
          tunnel: w1698 -> [w1710]
          frame #0 {
            n1158 = local write "Scan Speed (nm/s)"(w1707) -> ()
            n1159 = local write "Scan Range (nm)"(w1709) -> ()
            n1160 = local write "Step Size (nm)"(w1708) -> ()
          }
          frame #1 {
            n1161 = property on="Number of F/B Scans (AOD)" class="DigNum (strict)"("Val(Sgnl)"=w1710) -> ()  [unwired: 2 in, 2 out]
          }
        }
      }
      event "Trap 1 (ON/OFF)", "Trap 2 (ON/OFF)": Value Change {
        n1162 = event-data() -> ()  [unwired: 7 out]
        n1163 = flat-sequence {
          tunnel: [w1720] -> w1715
          tunnel: w1715 -> [w1735]
          tunnel: [w1721] -> w1711
          frame #0 {
            n1164 = local read "Trap 1 ON"() -> (w1720:bool)
          }
          frame #1 {
            n1165 = Exclusive Or(1:w1735, 2:"Trap 1 (ON/OFF)") -> (0:w1728:bool)
            n1166 = Select(t="on", s="Trap 2 (ON/OFF)", f="off") -> (s? t:f=w1727:string)
            n1167 = Select(t="on", s="Trap 1 (ON/OFF)", f="off") -> (s? t:f=w1723:string)
            n1168 = Build Array("trap 1 ", w1723) -> (w1722:string[])
            n1169 = Build Array("trap 2 " ("f"), w1727) -> (w1725:string[])
            n1170 = Select(t=w1722, s=w1728, f=w1725) -> (s? t:f=w1721:string[])
            n1171 = property on="Trap 1 ON" class="Bool (strict)"("Val(Sgnl)"="Trap 1 (ON/OFF)") -> ()  [unwired: 2 in, 2 out]
            n1172 = property on="Trap 2 ON" class="Bool (strict)"("Val(Sgnl)"="Trap 2 (ON/OFF)") -> ()  [unwired: 2 in, 2 out]
          }
        }
        n1173 = local read "Saving..."() -> (w1714:bool)
        n1174 = local read "Save Event Log?"() -> (w1713:bool)
        n1175 = And(x=w1714, y=w1713) -> (x .and. y?=w1712:bool)
        n1176 = case shown="True" w1712 {
          tunnel: w1711 -> [_ w1719]
          frame False {
          }
          frame True {
            n1177 = local read "Time (s)"() -> (w1716:dbl)
            n1178 = local read "log file ref"() -> (w1718:refnum<file>)
            n1179 = Concatenate Strings(w1719) -> (w1717:string)
            n1180 = call "write to event log.vi"("log file ref"=w1718, "time"=w1716, "input string"=w1717) -> ()  [unwired: 8 in]
          }
        }
      }
      event "DIO count 1 (ticks)", "DIO count 2 (ticks)", "DIO count 3 (ticks)", "Interlace", "Number Interlace Sets", "Not-Interlacing Set", "BD 1 Delay (ticks)", "BD 2 Delay (Ticks)", "Next trap write delay (ticks)", "XY phase ext loop method", "Amp switch delay 2", "BD 2 Delay (Ticks) 2", "BD 1 Delay (ticks) 2": Value Change {
        n1181 = event-data() -> ()  [unwired: 7 out]
        n1182 = local read "DIO count 3 (ticks)"() -> (w1751:u16)
        n1183 = local read "DIO count 1 (ticks)"() -> (w1753:u16)
        n1184 = local read "DIO count 2 (ticks)"() -> (w1752:u16)
        n1185 = To Unsigned Byte Integer(number="Not-Interlacing Set") -> (unsigned 8bit integer=w1742:u8)
        n1186 = Add(x=w1742, y=u8 1) -> (x+y=w1746:u8)
        n1187 = xnode "Read/Write Control"("FPGA VI Reference In"=w1736, "DIO count 1 (ticks)"=w1753, "DIO count 2 (ticks)"=w1752, "DIO count 3 (ticks)"=w1751, "Interlace ON/OFF"="Interlace", "Number Interlace Cycles"="Number Interlace Sets", "Interlace Off Parameters"=w1746, "BD 1 Delay (ticks)"="BD 1 Delay (ticks)", "BD 2 Delay (Ticks)"="BD 2 Delay (Ticks)", "Next trap write delay (ticks)"="Next trap write delay (ticks)", "XY phase ext loop method"="XY phase ext loop method") -> ("error out"=w1755:errorcluster)  [unwired: 1 in, 1 out]
        n1188 = Build Array(w1753, w1752, w1751) -> (w1744:u16[])
        n1189 = Split 1D Array(array=w1744, index="Number Interlace Sets") -> (first subarray=w1754:u16[])  [unwired: 1 out]
        n1190 = Index Array(array=w1744, index=w1742) -> (element=w1743:u16)
        n1191 = Add Array Elements(numeric array=w1754) -> (sum=w1748:u16)
        n1192 = Select(t=w1748, s="Interlace", f=w1743) -> (s? t:f=→"Total Counts (ticks)":u16)
      }
      event "Reset Feedback": Value Change {
        n1193 = event-data() -> ()  [unwired: 7 out]
        n1194 = Unbundle By Name("Reset Feedback") -> ("Set 1"=w1759:bool, "Set 2"=w1758:bool)
        n1195 = xnode "Read/Write Control"("FPGA VI Reference In"=w1756, "FB Reset Set 1"=w1759, "FB Reset Set 2"=w1758) -> ("error out"=w1757:errorcluster)  [unwired: 1 in, 1 out]
      }
      event "Trap Intensity PID Gains": Value Change {
        n1196 = event-data() -> ()  [unwired: 7 out]
        n1197 = Unbundle By Name("Trap Intensity PID Gains") -> ("proportional gain (Kc)"=w1764:i16, "integral gain (Kc*Ts/Ti)"=w1763:i16, "derivative gain (Kc*Td/Ts)"=w1762:i16)
        n1198 = xnode "Read/Write Control"("FPGA VI Reference In"=w1761, "P1"=w1764, "I1"=w1763, "D1"=w1762) -> ("error out"=w1766:errorcluster)  [unwired: 1 in, 1 out]
      }
      event "AI2 to Setpoint", "Setpoints (V)": Value Change {
        n1199 = event-data() -> ()  [unwired: 7 out]
        n1200 = xnode "Read/Write Control"("FPGA VI Reference In"=w1767) -> ("FPGA VI Reference Out"=w1770:T24, "error out"=w1769:errorcluster, "AI2 Y Sum Set 1"=w1777:i16, "AI2 Y Sum Set 2"=w1776:i16)  [unwired: 1 in]
        n1201 = Cluster To Array(cluster="AI2 to Setpoint") -> (array=w1780:bool[])
        n1202 = local read "AI2 (V)"() -> (w1778:cluster{"Set 1":dbl, "Set 2":dbl})
        n1203 = Or Array Elements(Boolean array=w1780) -> (logical OR=w1781:bool)
        n1204 = Bundle By Name(cluster=w1778, "Set 1"=w1777, "Set 2"=w1776) -> (w1775:cluster{"Set 1":dbl, "Set 2":dbl})
        n1205 = Divide(x=w1775, y=3276.7) -> (x/y=w1774:cluster{"Set 1":dbl, "Set 2":dbl})
        "AI2 (V)" <- w1774
        n1206 = case shown="True" w1781 {
          tunnel: [w1784 w1801] -> w1773
          tunnel: "AI2 to Setpoint" -> [_ w1797]
          tunnel: "Setpoints (V)" -> [w1785 w1800]
          tunnel: w1774 -> [_ w1794]
          frame False {
            n1207 = Multiply(x=3276.7, y=w1785) -> (x*y=w1786:cluster{"Set 1":dbl, "Set 2":dbl})
            n1208 = To Word Integer(number=w1786) -> (16bit integer=w1784:cluster{"Set 1":i16, "Set 2":i16})
          }
          frame True {
            n1209 = Unbundle By Name(w1794) -> ("Set 1"=w1793:dbl, "Set 2"=w1792:dbl)
            n1210 = Unbundle By Name(w1800) -> ("Set 1"=w1799:dbl, "Set 2"=w1798:dbl)
            n1211 = Unbundle By Name(w1797) -> ("Set 1"=w1796:bool, "Set 2"=w1795:bool)
            n1212 = Select(t=w1793, s=w1796, f=w1799) -> (s? t:f=w1791:dbl)
            n1213 = Select(t=w1792, s=w1795, f=w1798) -> (s? t:f=w1790:dbl)
            n1214 = Bundle By Name(cluster=w1800, "Set 1"=w1791, "Set 2"=w1790) -> (w1788:cluster{"Set 1":dbl, "Set 2":dbl})
            n1215 = local write "Setpoints (V)"(w1788) -> ()
            n1216 = Multiply(x=3276.7, y=w1788) -> (x*y=w1789:cluster{"Set 1":dbl, "Set 2":dbl})
            n1217 = To Word Integer(number=w1789) -> (16bit integer=w1801:cluster{"Set 1":i16, "Set 2":i16})
          }
        }
        n1218 = Unbundle By Name(w1773) -> ("Set 1"=w1772:i16, "Set 2"=w1771:i16)
        n1219 = xnode "Read/Write Control"("FPGA VI Reference In"=w1770, "error in"=w1769, "FB Setpoint Set 1"=w1772, "FB Setpoint Set 2"=w1771) -> ("error out"=w1768:errorcluster)  [unwired: 1 out]
      }
      event "+ phase (GI)", "- phase (GI)", "+ phase (GI) 2", "- phase (GI) 2", "+ phase (RI)", "- phase (RI)", "+ phase (Green FB)", "- phase (Green FB)", "- phase (BI AO)", "+ phase (BI AO)", "- phase (BI DO)", "+ phase (BI DO)": Value Change {
        n1220 = event-data() -> ()  [unwired: 7 out]
        n1221 = Or(x="+ phase (GI)", y="- phase (GI)") -> (x .or. y?=w1837:bool)
        n1222 = Negate(x="Phase adj. (GI)") -> (-x=w1842:i16)
        n1223 = Select(t=w1842, s="+ phase (GI)", f="Phase adj. (GI)") -> (s? t:f=w1841:i16)
        n1224 = Or(x="+ phase (GI) 2", y="- phase (GI) 2") -> (x .or. y?=w1828:bool)
        n1225 = Negate(x="Phase adj. (GI) 2") -> (-x=w1833:i16)
        n1226 = Select(t=w1833, s="+ phase (GI) 2", f="Phase adj. (GI) 2") -> (s? t:f=w1829:i16)
        n1227 = Negate(x="Phase adj. (RI)") -> (-x=w1827:i16)
        n1228 = Or(x="+ phase (RI)", y="- phase (RI)") -> (x .or. y?=w1823:bool)
        n1229 = Select(t=w1827, s="+ phase (RI)", f="Phase adj. (RI)") -> (s? t:f=w1822:i16)
        n1230 = Or(x="+ phase (Green FB)", y="- phase (Green FB)") -> (x .or. y?=w1816:bool)
        n1231 = Negate(x="Phase adj. (Green FB)") -> (-x=w1821:i16)
        n1232 = Select(t=w1821, s="+ phase (Green FB)", f="Phase adj. (Green FB)") -> (s? t:f=w1817:i16)
        n1233 = Negate(x="Phase adj. (BI AO)") -> (-x=w1815:i16)
        n1234 = Or(x="+ phase (BI AO)", y="- phase (BI AO)") -> (x .or. y?=w1805:bool)
        n1235 = Select(t=w1815, s="+ phase (BI AO)", f="Phase adj. (BI AO)") -> (s? t:f=w1807:i16)
        n1236 = Negate(x="Phase adj. (BI DO)") -> (-x=w1811:i16)
        n1237 = Or(x="+ phase (BI DO)", y="- phase (BI DO)") -> (x .or. y?=w1804:bool)